vi "Exercise2.1-FM Modulation Demo (Single Tone)-IQ - arctan.vi"() -> ()   [LabVIEW 2013]
uses:
  <vilib>/Analysis/NI_AALPro.lvlib
panel:
  in  "Mod. Freq.":dbl=2000.0 caption="Frequency"
  in  "WAV SR":dbl=44100.0 caption="dt"
  in  "LPF Cut-Off":dbl=60000.0 caption="Lower Cut-Off"
  in  "SNR (dB)":dbl(slide)=30.0 caption="Standard deviation" scale=-20.0..100.0
  out "Recovered Signal":dynamicdata(graph)=[{"t0"=timestamp(0 s since 1904-01-01), "dt"=1e-06, "Y"=array[100000 elements], "attributes"=variant("NI_ChannelName"=variant(string "Sine (Derivative (dX/dt))"), "NI_ExpIsRelativeTime"=variant(bool TRUE), "NI_ExpStartTimeStamp"=variant(timestamp timestamp(3676385695.5098023 s since 1904-01-01)), "NI_ExpTimeStamp"=variant(timestamp timestamp(3676385695.5098023 s since 1904-01-01)), "NI_ExpXDimension"=variant(string "t"), "NI_OriginalChannelName"=variant(string "Sine"))}]
  out "Baseband":dynamicdata(graph)=[{"t0"=timestamp(0 s since 1904-01-01), "dt"=1e-06, "Y"=array[100000 elements], "attributes"=variant("NI_ChannelName"=variant(string "Sine"), "NI_ExpIsRelativeTime"=variant(bool TRUE), "NI_ExpStartTimeStamp"=variant(timestamp timestamp(3676385695.5098023 s since 1904-01-01)), "NI_ExpTimeStamp"=variant(timestamp timestamp(3676385695.5098023 s since 1904-01-01)), "NI_ExpXDimension"=variant(string "t"))}]
  out "FM Spectrum":dynamicdata(graph)=[{"t0"=timestamp(0 s since 1904-01-01), "dt"=10.0, "Y"=array[50000 elements], "attributes"=variant("NI_ChannelName"=variant(string "Sine (Power Spectrum)"), "NI_ExpIsRelativeTime"=variant(bool TRUE), "NI_ExpStartTimeStamp"=variant(timestamp timestamp(3676385695.5098023 s since 1904-01-01)), "NI_ExpTimeStamp"=variant(timestamp timestamp(3676385695.5098023 s since 1904-01-01)), "NI_ExpXDimension"=variant(string "f"), "NI_OriginalChannelName"=variant(string "Sine"))}]
  out "FM Wave":dynamicdata(graph)=[{"t0"=timestamp(0 s since 1904-01-01), "dt"=1e-06, "Y"=array[100000 elements], "attributes"=variant("NI_ChannelName"=variant(string "Sine"), "NI_ExpIsRelativeTime"=variant(bool TRUE), "NI_ExpStartTimeStamp"=variant(timestamp timestamp(3676385695.5098023 s since 1904-01-01)), "NI_ExpTimeStamp"=variant(timestamp timestamp(3676385695.5098023 s since 1904-01-01)), "NI_ExpXDimension"=variant(string "t"))}, {"t0"=timestamp(0 s since 1904-01-01), "dt"=1e-06, "Y"=array[100000 elements], "attributes"=variant("NI_ChannelName"=variant(string "Sine (Integral (Sum[Xdt]))"), "NI_ExpIsRelativeTime"=variant(bool TRUE), "NI_ExpStartTimeStamp"=variant(timestamp timestamp(3676385695.5098023 s since 1904-01-01)), "NI_ExpTimeStamp"=variant(timestamp timestamp(3676385695.5098023 s since 1904-01-01)), "NI_ExpXDimension"=variant(string "t"), "NI_OriginalChannelName"=variant(string "Sine"))}]
  in  "Carrier Amp.":dbl=1.0 caption="Amplitude"
  in  "stop":bool
  in  "Frequency Deviation":dbl(slide)=200.0 scale=0.0..75000.0
  in  "Carrier Freq.":dbl=100000.0 caption="Frequency"
  # "正交解调低通滤波器的截止频率不应设置为基带信号频率，WBFM调频之后带宽增加！"
  # "Frequency Modulation"
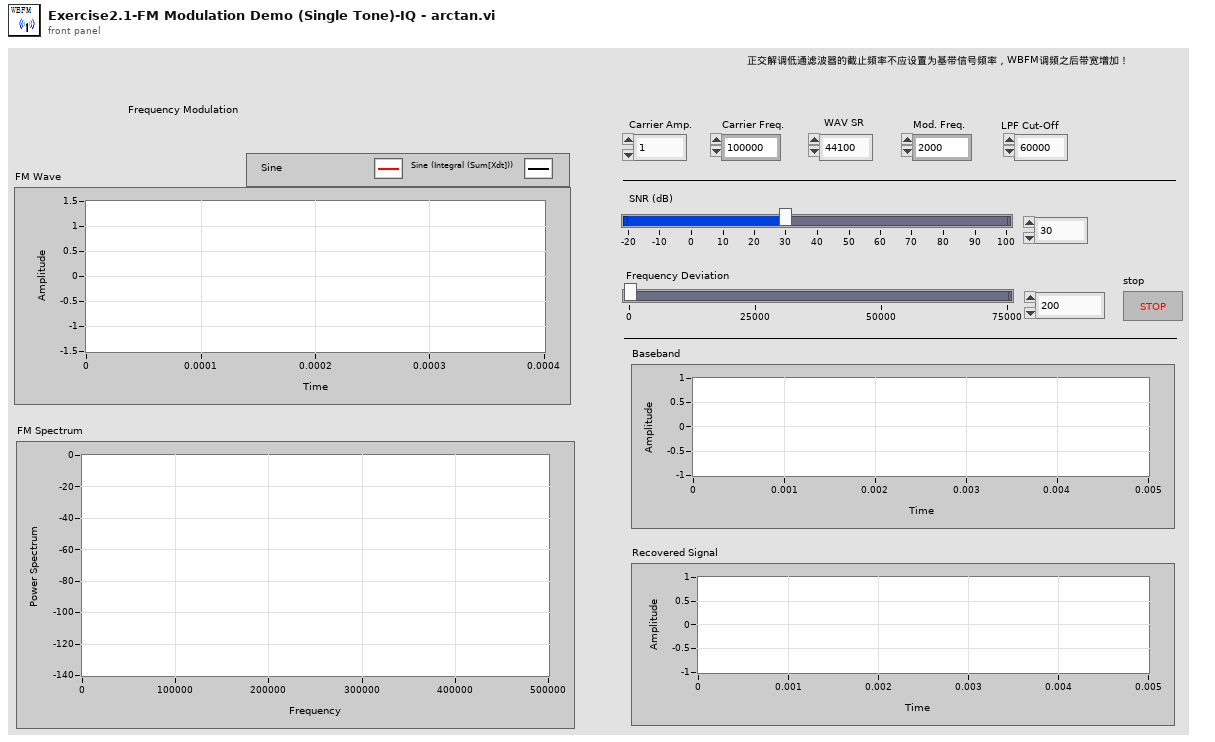
[diagram p1: front panel]
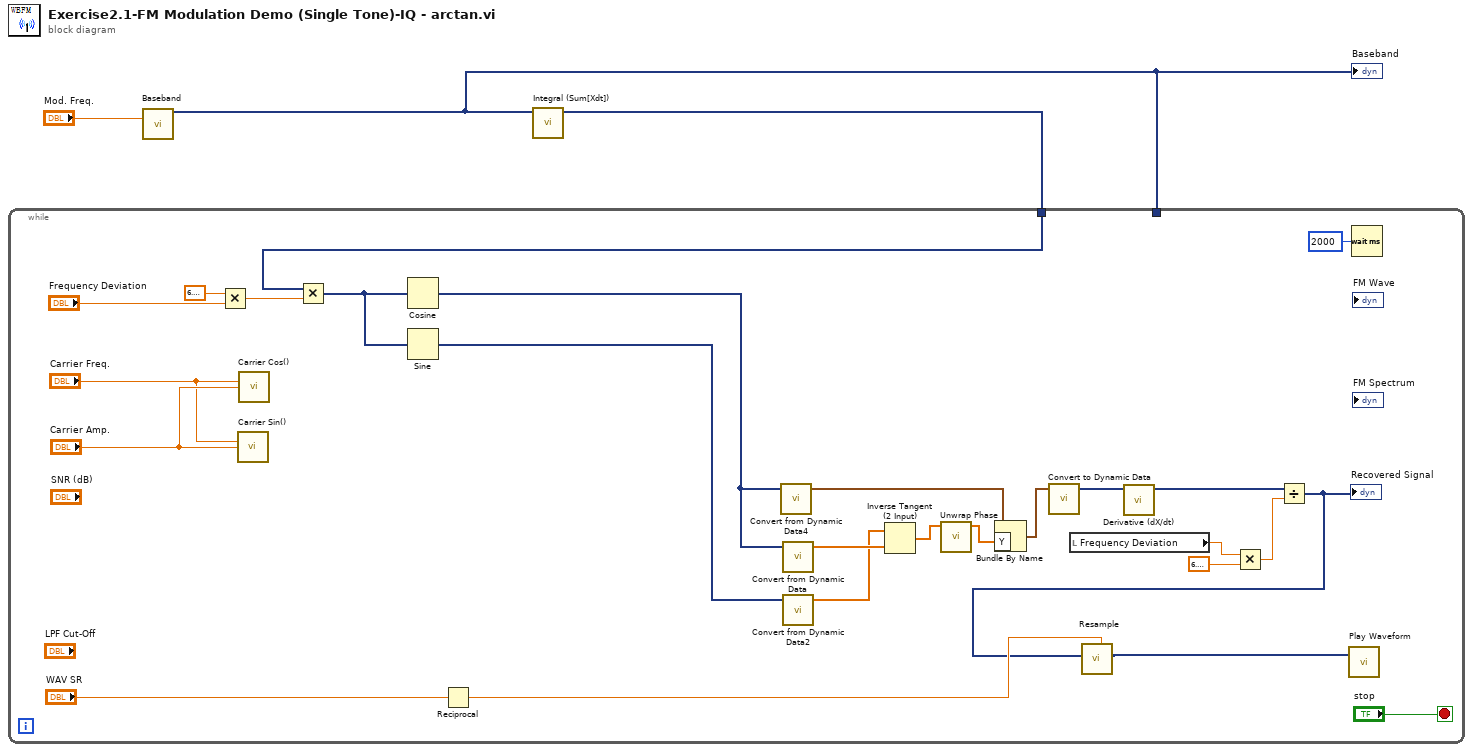
[diagram p0: block diagram]
diagram:
  n1 = call "Baseband"("Frequency"="Mod. Freq.") -> ("Sine"=w2:dynamicdata)  [unwired: 13 in, 1 out]
  "Baseband" <- w2
  n2 = call "Integral (Sum[Xdt])"("Signals"=w2) -> ("Result"=w3:dynamicdata)  [unwired: 5 in, 1 out]
  n3 = while {
    tunnel: w3 -> [w19]
    tunnel: w2 -> [_]
    stop <- "stop" stop-if-true
    n4 = Multiply(x=6.283185307179586, y="Frequency Deviation") -> (x*y=w22:dbl)
    n5 = call "Carrier Sin()"("Frequency"="Carrier Freq.", "Amplitude"="Carrier Amp.") -> ()  [unwired: 12 in, 2 out]
    n6 = call "Carrier Cos()"("Frequency"="Carrier Freq.", "Amplitude"="Carrier Amp.") -> ()  [unwired: 12 in, 2 out]
    n7 = Multiply ("Multiplier")(x=w19, y=w22) -> (x*y=w21:dynamicdata)
    n8 = Cosine(x=w21) -> (cos(x)=w7:dynamicdata)
    n9 = Sine(x=w21) -> (sin(x)=w4:dynamicdata)
    n10 = Reciprocal(x="WAV SR") -> (1/x=w18:dbl)
    n11 = call "Convert from Dynamic Data4"("Dynamic Data Type"=w7) -> ("Waveform"=w16:waveform(dbl))  [unwired: 3 in]
    n12 = call "Convert from Dynamic Data"("Dynamic Data Type"=w7) -> ("Array"=w6:dbl[])  [unwired: 3 in]
    n13 = call "Convert from Dynamic Data2"("Dynamic Data Type"=w4) -> ("Array"=w5:dbl[])  [unwired: 3 in]
    n14 = Inverse Tangent (2 Input)(1:w6, 2:w5) -> (0:w20:dbl[])
    n15 = call <vilib>:"Unwrap Phase.vi"("Phase"=w20) -> ("Unwrapped Phase"=w17:dbl[])  [unwired: 9 in, 1 out]
    n16 = Bundle By Name(cluster=w16, "Y"=w17) -> (w15:waveform(dbl))
    n17 = call "Convert to Dynamic Data"("Waveform"=w15) -> ("Dynamic Data Type"=w14:dynamicdata)  [unwired: 3 in]
    n18 = local read "Frequency Deviation"() -> (w12:dbl)
    n19 = call "Derivative (dX/dt)"("Signals"=w14) -> ("Result"=w10:dynamicdata)  [unwired: 5 in, 1 out]
    n20 = Multiply(x=w12, y=6.283185307179586) -> (x*y=w8:dbl)
    n21 = Divide(x=w10, y=w8) -> (x/y=w9:dynamicdata)
    "Recovered Signal" <- w9
    n22 = call "Resample"("dt"=w18, "Signals"=w9) -> ("Resampled Signals"=w13:dynamicdata)  [unwired: 7 in, 2 out]
    n23 = call "Play Waveform"("Data"=w13) -> ()  [unwired: 18 in, 1 out]
    n24 = Wait (ms)(milliseconds to wait=u32 2000) -> ()  [unwired: 1 out]
  }
